vi "UHR-Fleezers Control (host) - 12.7d.vi"() -> ()   [LabVIEW 2012] (continued)
      }
      event "Load parameters": Value Change {
        n400 = event-data() -> ()  [unwired: 7 out]
        n401 = property on="Saved AOD Raster Scan Parameter Sets" class="Arr (strict)"() -> ("Index Values"=w577:u32[])  [unwired: 2 in, 2 out]
        n402 = Index Array(array=w577, index=0) -> (element=w574:u32)
        n403 = local write "Load parameters"(FALSE ("Load parameters")) -> ()
        n404 = Index Array(array="Saved AOD Raster Scan Parameter Sets", index=w574) -> (element=w573:T28)
        n405 = Unbundle By Name(w573) -> ("Scan Range AOD (nm) 2"=w572:dbl, "Step Size AOD (nm) 2"=w571:dbl, "Scan Speed AOD (nm/s) 2"=w570:dbl, "Number of scans (AOD) 2"=w569:u16)
        n406 = flat-sequence {
          tunnel: w572 -> [w580]
          tunnel: w571 -> [w579]
          tunnel: w570 -> [w578]
          tunnel: w569 -> [w581]
          frame #0 {
            n407 = local write "Scan Speed (nm/s)"(w578) -> ()
            n408 = local write "Scan Range (nm)"(w580) -> ()
            n409 = local write "Step Size (nm)"(w579) -> ()
          }
          frame #1 {
            n410 = property on="Number of F/B Scans (AOD)" class="DigNum (strict)"("Val(Sgnl)"=w581) -> ()  [unwired: 2 in, 2 out]
          }
        }
      }
      event "Trap 1 (ON/OFF)", "Trap 2 (ON/OFF)": Value Change {
        n411 = event-data() -> ()  [unwired: 7 out]
        n412 = property on="Trap 2 ON" class="Bool (strict)"("Val(Sgnl)"="Trap 2 (ON/OFF)") -> ()  [unwired: 2 in, 2 out]
        n413 = property on="Trap 1 ON" class="Bool (strict)"("Val(Sgnl)"="Trap 1 (ON/OFF)") -> ()  [unwired: 2 in, 2 out]
      }
      event "DIO count 1 (ticks)", "DIO count 2 (ticks)", "DIO count 3 (ticks)", "Interlace", "Number Interlace Sets", "Not-Interlacing Set", "BD 1 Delay (ticks)", "BD 2 Delay (Ticks)", "Next trap write delay (ticks)", "XY phase ext loop method", "Amp switch delay 2", "BD 2 Delay (Ticks) 2", "BD 1 Delay (ticks) 2": Value Change {
        n414 = event-data() -> ()  [unwired: 7 out]
        n415 = local read "DIO count 3 (ticks)"() -> (w602:u16)
        n416 = local read "DIO count 1 (ticks)"() -> (w604:u16)
        n417 = local read "DIO count 2 (ticks)"() -> (w603:u16)
        n418 = To Unsigned Byte Integer(number="Not-Interlacing Set") -> (unsigned 8bit integer=w593:u8)
        n419 = Add(x=w593, y=u8 1) -> (x+y=w597:u8)
        n420 = xnode "Read/Write Control"("FPGA VI Reference In"=w584, "DIO count 1 (ticks)"=w604, "DIO count 2 (ticks)"=w603, "DIO count 3 (ticks)"=w602, "Interlace ON/OFF"="Interlace", "Number Interlace Cycles"="Number Interlace Sets", "Interlace Off Parameters"=w597, "BD 1 Delay (ticks)"="BD 1 Delay (ticks)", "BD 2 Delay (Ticks)"="BD 2 Delay (Ticks)", "Next trap write delay (ticks)"="Next trap write delay (ticks)", "XY phase ext loop method"="XY phase ext loop method", "Amp switch delay 2"="Amp switch delay 2", "BD 2 Delay (Ticks) 2"="BD 2 Delay (Ticks) 2", "BD 1 Delay (ticks) 2"="BD 1 Delay (ticks) 2") -> ("error out"=w606:errorcluster)  [unwired: 1 in, 1 out]
        n421 = Build Array(w604, w603, w602) -> (w595:u16[])
        n422 = Split 1D Array(array=w595, index="Number Interlace Sets") -> (first subarray=w605:u16[])  [unwired: 1 out]
        n423 = Index Array(array=w595, index=w593) -> (element=w594:u16)
        n424 = Add Array Elements(numeric array=w605) -> (sum=w599:u16)
        n425 = Select(t=w599, s="Interlace", f=w594) -> (s? t:f=→"Total Counts (ticks)":u16)
      }
      event "Reset Feedback": Value Change {
        n426 = event-data() -> ()  [unwired: 7 out]
        n427 = Unbundle By Name("Reset Feedback") -> ("Set 1"=w610:bool, "Set 2"=w609:bool)
        n428 = xnode "Read/Write Control"("FPGA VI Reference In"=w607, "FB Reset Set 1"=w610, "FB Reset Set 2"=w609) -> ("error out"=w608:errorcluster)  [unwired: 1 in, 1 out]
      }
      event "Trap Intensity PID Gains": Value Change {
        n429 = event-data() -> ()  [unwired: 7 out]
        n430 = Unbundle By Name("Trap Intensity PID Gains") -> ("proportional gain (Kc)"=w615:i16, "integral gain (Kc*Ts/Ti)"=w614:i16, "derivative gain (Kc*Td/Ts)"=w613:i16)
        n431 = xnode "Read/Write Control"("FPGA VI Reference In"=w612, "P1"=w615, "I1"=w614, "D1"=w613) -> ("error out"=w617:errorcluster)  [unwired: 1 in, 1 out]
      }
      event "AI2 to Setpoint", "Setpoints (V)": Value Change {
        n432 = event-data() -> ()  [unwired: 7 out]
        n433 = xnode "Read/Write Control"("FPGA VI Reference In"=w618) -> ("FPGA VI Reference Out"=w621:T20, "error out"=w620:errorcluster, "AI2 Y Sum Set 1"=w628:i16, "AI2 Y Sum Set 2"=w627:i16)  [unwired: 1 in]
        n434 = Cluster To Array(cluster="AI2 to Setpoint") -> (array=w631:bool[])
        n435 = local read "AI2 (V)"() -> (w629:cluster{"Set 1":dbl, "Set 2":dbl})
        n436 = Or Array Elements(Boolean array=w631) -> (logical OR=w632:bool)
        n437 = Bundle By Name(cluster=w629, "Set 1"=w628, "Set 2"=w627) -> (w626:cluster{"Set 1":dbl, "Set 2":dbl})
        n438 = Divide(x=w626, y=3276.7) -> (x/y=w625:cluster{"Set 1":dbl, "Set 2":dbl})
        "AI2 (V)" <- w625
        n439 = case shown="True" w632 {
          tunnel: [w635 w652] -> w624
          tunnel: "AI2 to Setpoint" -> [_ w648]
          tunnel: "Setpoints (V)" -> [w636 w651]
          tunnel: w625 -> [_ w645]
          frame False {
            n440 = Multiply(x=3276.7, y=w636) -> (x*y=w637:cluster{"Set 1":dbl, "Set 2":dbl})
            n441 = To Word Integer(number=w637) -> (16bit integer=w635:cluster{"Set 1":i16, "Set 2":i16})
          }
          frame True {
            n442 = Unbundle By Name(w645) -> ("Set 1"=w644:dbl, "Set 2"=w643:dbl)
            n443 = Unbundle By Name(w651) -> ("Set 1"=w650:dbl, "Set 2"=w649:dbl)
            n444 = Unbundle By Name(w648) -> ("Set 1"=w647:bool, "Set 2"=w646:bool)
            n445 = Select(t=w644, s=w647, f=w650) -> (s? t:f=w642:dbl)
            n446 = Select(t=w643, s=w646, f=w649) -> (s? t:f=w641:dbl)
            n447 = Bundle By Name(cluster=w651, "Set 1"=w642, "Set 2"=w641) -> (w639:cluster{"Set 1":dbl, "Set 2":dbl})
            n448 = local write "Setpoints (V)"(w639) -> ()
            n449 = Multiply(x=3276.7, y=w639) -> (x*y=w640:cluster{"Set 1":dbl, "Set 2":dbl})
            n450 = To Word Integer(number=w640) -> (16bit integer=w652:cluster{"Set 1":i16, "Set 2":i16})
          }
        }
        n451 = Unbundle By Name(w624) -> ("Set 1"=w623:i16, "Set 2"=w622:i16)
        n452 = xnode "Read/Write Control"("FPGA VI Reference In"=w621, "error in"=w620, "FB Setpoint Set 1"=w623, "FB Setpoint Set 2"=w622) -> ("error out"=w619:errorcluster)  [unwired: 1 out]
      }
      event "+ phase (GI)", "- phase (GI)", "+ phase (GI) 2", "- phase (GI) 2", "+ phase (RI)", "- phase (RI)", "+ phase (Green FB)", "- phase (Green FB)": Value Change {
        n453 = event-data() -> ()  [unwired: 7 out]
        n454 = Or(x="+ phase (GI)", y="- phase (GI)") -> (x .or. y?=w688:bool)
        n455 = Negate(x="Phase adj. (GI)") -> (-x=w693:i16)
        n456 = Select(t=w693, s="+ phase (GI)", f="Phase adj. (GI)") -> (s? t:f=w692:i16)
        n457 = Or(x="+ phase (GI) 2", y="- phase (GI) 2") -> (x .or. y?=w679:bool)
        n458 = Negate(x="Phase adj. (GI) 2") -> (-x=w684:i16)
        n459 = Select(t=w684, s="+ phase (GI) 2", f="Phase adj. (GI) 2") -> (s? t:f=w680:i16)
        n460 = Negate(x="Phase adj. (RI)") -> (-x=w678:i16)
        n461 = Or(x="+ phase (RI)", y="- phase (RI)") -> (x .or. y?=w674:bool)
        n462 = Select(t=w678, s="+ phase (RI)", f="Phase adj. (RI)") -> (s? t:f=w673:i16)
        n463 = Or(x="+ phase (Green FB)", y="- phase (Green FB)") -> (x .or. y?=w667:bool)
        n464 = Negate(x="Phase adj. (Green FB)") -> (-x=w672:i16)
        n465 = Select(t=w672, s="+ phase (Green FB)", f="Phase adj. (Green FB)") -> (s? t:f=w668:i16)
        n466 = Negate(x="Phase adj. (BI AO)") -> (-x=w666:i16)
        n467 = Or(x="+ phase (BI AO)", y="- phase (BI AO)") -> (x .or. y?=w656:bool)
        n468 = Select(t=w666, s="+ phase (BI AO)", f="Phase adj. (BI AO)") -> (s? t:f=w658:i16)
        n469 = Negate(x="Phase adj. (BI DO)") -> (-x=w662:i16)
        n470 = Or(x="+ phase (BI DO)", y="- phase (BI DO)") -> (x .or. y?=w655:bool)
        n471 = Select(t=w662, s="+ phase (BI DO)", f="Phase adj. (BI DO)") -> (s? t:f=w657:i16)
        n472 = xnode "Read/Write Control"("FPGA VI Reference In"=w654, "Phase count adjustment (GI)"=w692, "Phase count adjustment (GI) 2"=w680, "Phase count adjustment (RI)"=w673, "Phase count adjustment (Green FB)"=w668, "Phase count adjustment (BI AO)"=w658, "Phase count adjustment (BI D)"=w657) -> ("FPGA VI Reference Out"=w690:T20, "error out"=w691:errorcluster)  [unwired: 1 in]
        n473 = xnode "Read/Write Control"("FPGA VI Reference In"=w690, "error in"=w691, "+ phase (GI)"=w688, "+ phase (GI) 2"=w679, "+ phase (RI)"=w674, "+ phase (Green FB)"=w667, "+ phase (BI AO)"=w656, "+ phase (BI D)"=w655) -> ("error out"=w689:errorcluster)  [unwired: 1 out]
      }
      event "Green Laser ON/OFF", "Red Laser ON/OFF", "Blue Laser ON/OFF": Value Change {
        # "This loop shouldn't be initialized.  The main 'laser ON' settings should dominate and set the others."
        n474 = event-data() -> ()  [unwired: 7 out]
        n475 = property on="Red Laser ON" class="Bool (strict)"("Val(Sgnl)"="Red Laser ON/OFF") -> ()  [unwired: 2 in, 2 out]
        n476 = property on="Blue Laser ON" class="Bool (strict)"("Val(Sgnl)"="Blue Laser ON/OFF") -> ()  [unwired: 2 in, 2 out]
        n477 = property on="Green Laser ON" class="Bool (strict)"("Val(Sgnl)"="Green Laser ON/OFF") -> ()  [unwired: 2 in, 2 out]
      }
      event "Laser interlacing mode", "Green Laser ON", "Red Laser ON", "Blue Laser ON": Value Change {
        n478 = event-data() -> ()  [unwired: 7 out]
        n479 = local write "Green Laser ON/OFF"("Green Laser ON") -> ()
        n480 = local write "Blue Laser ON/OFF"("Blue Laser ON") -> ()
        n481 = local write "Red Laser ON/OFF"("Red Laser ON") -> ()
        n482 = case shown="True" "Green Laser ON" {
          tunnel: "Laser interlacing mode" -> [_ w729]
          tunnel: [enum32{"Laser ON", "Laser OFF", "Interlace"}."Laser OFF" ("Green laser mode") w729] -> w707
          tunnel: [FALSE w725] -> w706
          frame False {
          }
          frame True {
            n483 = local read "Green FB On/Off"() -> (w726:bool)
            n484 = Equal?(x=w729, y=enum32{"Laser ON", "Laser OFF", "Interlace"}."Interlace") -> (x = y?=w727:bool)
            n485 = And(x=w727, y=w726) -> (x .and. y?=w725:bool)
          }
        }
        n486 = case shown="True" "Red Laser ON" {
          tunnel: "Laser interlacing mode" -> [_ w722]
          tunnel: [enum32{"Laser ON", "Laser OFF", "Interlace"}."Laser OFF" ("Green laser mode") w722] -> w703
          tunnel: [FALSE w718] -> w702
          frame False {
          }
          frame True {
            n487 = local read "Red FB On/Off"() -> (w719:bool)
            n488 = Equal?(x=w722, y=enum32{"Laser ON", "Laser OFF", "Interlace"}."Interlace") -> (x = y?=w720:bool)
            n489 = And(x=w720, y=w719) -> (x .and. y?=w718:bool)
          }
        }
        n490 = case shown="True" "Blue Laser ON" {
          tunnel: "Laser interlacing mode" -> [_ w713]
          tunnel: [enum32{"Laser ON", "Laser OFF", "Interlace"}."Laser OFF" ("Green laser mode") w713] -> w699
          tunnel: [FALSE w711] -> w698
          frame False {
          }
          frame True {
            n491 = local read "Blue FB On/Off"() -> (w712:bool)
            n492 = Equal?(x=w713, y=enum32{"Laser ON", "Laser OFF", "Interlace"}."Interlace") -> (x = y?=w714:bool)
            n493 = And(x=w714, y=w712) -> (x .and. y?=w711:bool)
          }
        }
        n494 = xnode "Read/Write Control"("FPGA VI Reference In"=w697, "Operating Mode"=w707, "Operating Mode 2"=w707, "Green FB On/Off"=w706, "Red Laser Operating Mode"=w703, "RI Operating Mode 2"=w703, "Red FB On/Off"=w702, "BI Operating Mode (AO)"=w699, "Blue Laser Operating Mode (D)"=w699, "Blue FB On/Off"=w698) -> ("error out"=w708:errorcluster)  [unwired: 1 in, 1 out]
      }
      event "Invert laser interlacing": Value Change {
        n495 = event-data() -> ()  [unwired: 7 out]
        n496 = xnode "Read/Write Control"("FPGA VI Reference In"=w730, "Invert GI"="Invert laser interlacing", "Invert GI 2"="Invert laser interlacing", "Invert RI"="Invert laser interlacing", "Invert RI 2"="Invert laser interlacing", "Invert BI (AO)"="Invert laser interlacing", "Invert BI (D)"="Invert laser interlacing") -> ("error out"=w732:errorcluster)  [unwired: 1 in, 1 out]
      }
      event "Green FB Setpoint (mV)", "Green FB Gains", "Green FB On/Off", "Green Intensity % (FB OFF)", "Green int current ON count adj": Value Change {
        n497 = event-data() -> ()  [unwired: 7 out]
        n498 = local read "Green FB Setpoint (mV)"() -> (w744:dbl)
        n499 = Multiply(x=w744, y=3.2767) -> (x*y=w743:dbl)
        n500 = local read "Green Intensity % (FB OFF)"() -> (w747:dbl)
        n501 = Multiply(x=w747, y=655.35) -> (x*y=w748:dbl)
        n502 = To Unsigned Word Integer(number=w748) -> (unsigned 16bit integer=w746:u16)
        n503 = local read "Green int current ON count adj"() -> (w750:u32)
        n504 = local read "Laser interlacing mode"() -> (w740:enum32{"Laser ON", "Laser OFF", "Interlace"})
        n505 = local read "Green FB Gains"() -> (w737:T9)
        n506 = local read "Green Laser ON"() -> (w741:bool)
        n507 = local read "Green FB On/Off"() -> (w751:bool)
        n508 = Equal?(x=w740, y=enum32{"Laser ON", "Laser OFF", "Interlace"}."Interlace") -> (x = y?=w738:bool)
        n509 = Unbundle By Name(w737) -> ("proportional gain (Kc)"=w736:i16, "integral gain (Kc*Ts/Ti)"=w735:i16, "derivative gain (Kc*Td/Ts)"=w734:i16)
        n510 = Compound Arithmetic op=AND(w738, w751, w741) -> (w742:bool)
        n511 = xnode "Read/Write Control"("FPGA VI Reference In"=w733, "Green FB Setpoint"=w743, "Green FB On/Off"=w742, "Current Out"=w746, "Green int current ON count adj"=w750, "P3"=w736, "I3"=w735, "D3"=w734) -> ("error out"=w752:errorcluster)  [unwired: 1 in, 1 out]
      }
      event "Blue FB Setpoint (mV)", "Blue FB Gains", "Blue FB On/Off", "Blue Intensity % (FB OFF)", "Blue int AO ON count adjust": Value Change {
        # "16 bit analog out"
        n512 = event-data() -> ()  [unwired: 7 out]
        n513 = Multiply(x="Blue FB Setpoint (mV)", y=3.2767) -> (x*y=w767:dbl)
        n514 = Multiply(x="Blue Intensity % (FB OFF)", y=655.35) -> (x*y=w770:dbl)
        n515 = To Unsigned Word Integer(number=w770) -> (unsigned 16bit integer=w769:u16)
        n516 = local read "Laser interlacing mode"() -> (w765:enum32{"Laser ON", "Laser OFF", "Interlace"})
        n517 = Unbundle By Name("Blue FB Gains") -> ("proportional gain (Kc)"=w762:i16, "integral gain (Kc*Ts/Ti)"=w761:i16, "derivative gain (Kc*Td/Ts)"=w760:i16)
        n518 = local read "Blue Laser ON"() -> (w754:bool)
        n519 = Equal?(x=w765, y=enum32{"Laser ON", "Laser OFF", "Interlace"}."Interlace") -> (x = y?=w763:bool)
        n520 = Compound Arithmetic op=AND(w763, "Blue FB On/Off", w754) -> (w766:bool)
        n521 = xnode "Read/Write Control"("FPGA VI Reference In"=w753, "Blue FB Setpoint"=w767, "Blue FB On/Off"=w766, "BI Current Out"=w769, "Blue current ON count adj (AO)"="Blue int AO ON count adjust", "P5"=w762, "I5"=w761, "D5"=w760) -> ("error out"=w772:errorcluster)  [unwired: 1 in, 1 out]
      }
      event "Red FB Setpoint (mV)", "Red FB Gains", "Red FB On/Off", "Red Intensity % (FB OFF)": Value Change {
        n522 = event-data() -> ()  [unwired: 7 out]
        n523 = local read "Red FB Setpoint (mV)"() -> (w785:dbl)
        n524 = Multiply(x=w785, y=3.2767) -> (x*y=w784:dbl)
        n525 = local read "Red Intensity % (FB OFF)"() -> (w774:dbl)
        n526 = Multiply(x=w774, y=655.35) -> (x*y=w788:dbl)
        n527 = To Unsigned Word Integer(number=w788) -> (unsigned 16bit integer=w787:u16)
        n528 = local read "Laser interlacing mode"() -> (w781:enum32{"Laser ON", "Laser OFF", "Interlace"})
        n529 = local read "Red FB Gains"() -> (w778:T9)
        n530 = local read "Red Laser ON"() -> (w782:bool)
        n531 = local read "Red FB On/Off"() -> (w790:bool)
        n532 = Equal?(x=w781, y=enum32{"Laser ON", "Laser OFF", "Interlace"}."Interlace") -> (x = y?=w779:bool)
        n533 = Unbundle By Name(w778) -> ("proportional gain (Kc)"=w777:i16, "integral gain (Kc*Ts/Ti)"=w776:i16, "derivative gain (Kc*Td/Ts)"=w775:i16)
        n534 = Compound Arithmetic op=AND(w779, w790, w782) -> (w783:bool)
        n535 = xnode "Read/Write Control"("FPGA VI Reference In"=w773, "Red FB Setpoint"=w784, "Red FB On/Off"=w783, "RI Current Out"=w787, "P4"=w777, "I4"=w776, "D4"=w775) -> ("error out"=w791:errorcluster)  [unwired: 1 in, 1 out]
      }
      event "+ phase (APD 1 Gate)", "- phase (APD 1 Gate)", "+ phase (APD 2 Gate)", "- phase (APD 2 Gate)", "+ phase (APD 3 Gate)", "- phase (APD 3 Gate)", "+ phase (APD Acq)", "- phase (APD Acq)": Value Change {
        n536 = event-data() -> ()  [unwired: 7 out]
        n537 = local read "Phase Adj. (APD 1 Gate)"() -> (w812:i16)
        n538 = Or(x="- phase (APD 1 Gate)", y="+ phase (APD 1 Gate)") -> (x .or. y?=w814:bool)
        n539 = Negate(x=w812) -> (-x=w819:i16)
        n540 = Select(t=w819, s="+ phase (APD 1 Gate)", f=w812) -> (s? t:f=w818:i16)
        n541 = local read "Phase Adj. (APD 2 Gate)"() -> (w809:i16)
        n542 = Or(x="- phase (APD 2 Gate)", y="+ phase (APD 2 Gate)") -> (x .or. y?=w807:bool)
        n543 = Negate(x=w809) -> (-x=w811:i16)
        n544 = Select(t=w811, s="+ phase (APD 2 Gate)", f=w809) -> (s? t:f=w808:i16)
        n545 = Negate(x="Phase Adj. (APD 3 Gate)") -> (-x=w806:i16)
        n546 = Or(x="- phase (APD 3 Gate)", y="+ phase (APD 3 Gate)") -> (x .or. y?=w802:bool)
        n547 = Select(t=w806, s="+ phase (APD 3 Gate)", f="Phase Adj. (APD 3 Gate)") -> (s? t:f=w803:i16)
        n548 = local read "Phase Adj. (APD Acq)"() -> (w800:i16)
        n549 = Or(x="- phase (APD Acq)", y="+ phase (APD Acq)") -> (x .or. y?=w798:bool)
        n550 = Negate(x=w800) -> (-x=w801:i16)
        n551 = Select(t=w801, s="+ phase (APD Acq)", f=w800) -> (s? t:f=w799:i16)
        n552 = xnode "Read/Write Control"("FPGA VI Reference In"=w792, "Phase count adjustment (APD 1 Gate)"=w818, "Phase count adjustment (APD 2 Gate)"=w808, "Phase count adjustment (APD 3 Gate)"=w803, "Phase Count Adjustment (APD Acq)"=w799) -> ("FPGA VI Reference Out"=w816:T20, "error out"=w817:errorcluster)  [unwired: 1 in]
        n553 = xnode "Read/Write Control"("FPGA VI Reference In"=w816, "error in"=w817, "+ phase (APD 1 Gate)"=w814, "+ phase (APD 2 Gate)"=w807, "+ phase (APD 3 Gate)"=w802, "+ phase (APD Acq)"=w798) -> ("error out"=w815:errorcluster)  [unwired: 1 out]
      }
      event "Invert APD Gate", "APD Gate ON Count", "APD Gate OFF Count", "APD Gate", "APD Integration Time (s)", "APD AO Scale Factor", "Duty Frequency (ON 1/N cycles)", "Interlace ON count", "Interlace OFF count": Value Change {
        n554 = event-data() -> ()  [unwired: 7 out]
        n555 = Add(x="Interlace ON count", y="Interlace OFF count") -> (x+y=w826:u16)
        n556 = Add(x="APD Gate ON Count", y="APD Gate OFF Count") -> (x+y=w837:u16)
        n557 = Multiply(x="Duty Frequency (ON 1/N cycles)", y=w826) -> (x*y=w822:u16)
        "Green AI Count" <- w822
        "Red AI Count" <- w822
        "Blue AI Count" <- w822
        n558 = Subtract(x=w822, y="Interlace ON count") -> (x-y=w825:u16)
        n559 = Multiply(x=w837, y="Duty Frequency (ON 1/N cycles)") -> (x*y=w836:u16)
        n560 = Subtract(x=w836, y="APD Gate ON Count") -> (x-y=w835:u16)
        n561 = local read "DMA Update Period (s)"() -> (w838:dbl)
        n562 = Multiply(x="APD Integration Time (s)", y=40000000.0) -> (x*y=w842:dbl)
        n563 = Reciprocal(x="APD Integration Time (s)") -> (1/x=→"APD Acq Rate (Hz)":dbl)
        n564 = To Unsigned Long Integer(number=w842) -> (unsigned 32bit integer=w828:u32)
        "APD Int. Count" <- w828
        n565 = local read "Number of APDs"() -> (w821:u8)
        n566 = Divide(x=w838, y="APD Integration Time (s)") -> (x/y=w840:dbl)
        n567 = Multiply(x=w821, y=w840) -> (x*y=w839:dbl)
        n568 = local write "APD Samples/FIFO Acq."(w840) -> ()
        n569 = local write "APD Elements/DMA read"(w839) -> ()
        n570 = xnode "Read/Write Control"("FPGA VI Reference In"=w820, "Invert APD Gate"="Invert APD Gate", "APD Gate ON Count"="APD Gate ON Count", "APD Gate OFF Count"=w835, "APD Acq Rate Count"=w828, "APD Gate Operating Mode"="APD Gate", "APD AO scale factor"="APD AO Scale Factor", "Green interlace ON count"="Interlace ON count", "Green interlace OFF count"=w825, "Green interlace ON count 2"="Interlace ON count", "Green interlace OFF count 2"=w825, "Green FB Count"=w822, "Red interlace ON count"="Interlace ON count", "Red interlace OFF count"="Interlace OFF count", "Blue ON count (AO)"="Interlace ON count", "Blue OFF count (AO)"="Interlace OFF count", "Blue interlace OFF count (D)"="Interlace OFF count", "Blue interlace ON count (D)"="Interlace ON count") -> ("error out"=w844:errorcluster)  [unwired: 1 in, 1 out]
      }
      event "Neg. TTrig FPGA": Value Change {
        n571 = event-data() -> ()  [unwired: 7 out]
        n572 = xnode "Read/Write Control"("FPGA VI Reference In"=w845, "TTrig Negate Pos"="Neg. TTrig FPGA") -> ()  [unwired: 1 in, 2 out]
      }
      event "Test ttrig": Value Change {
        n573 = event-data() -> ()  [unwired: 7 out]
        n574 = xnode "Read/Write Control"("FPGA VI Reference In"=w847, "TTrig?"=TRUE) -> ("error out"=w849:errorcluster)  [unwired: 1 in, 1 out]
      }
      event "Number of F/B Scans (AOD)", "Scan Speed (nm/s)", "Scan BD", "Initial delta (MHz)", "Step Size (nm)", "Scan Range (nm)": Value Change {
        w913 = 123.0  # AOM cal (nm/MHz)
        n575 = event-data() -> ()  [unwired: 7 out]
        n576 = local read "BD 1 Frequency 1 (MHz)"() -> (w896:dbl)
        n577 = local read "AOM X Cal (nm/MHz)"() -> (w888:dbl)
        n578 = local read "X RF Frequency Limits (MHz)"() -> (w900:T16)
        n579 = local read "Y RF Frequency Limits (MHz)"() -> (w897:T16)
        n580 = local read "BD 2 Frequency 1 (MHz)"() -> (w902:dbl)
        n581 = Negate(x="Scan Range (nm)") -> (-x=w866:dbl)
        n582 = Divide(x=w866, y=w888) -> (x/y=w870:dbl)
        n583 = Select(t=w900, s="Scan BD", f=w897) -> (s? t:f=w899:T16)
        n584 = Select(t=w896, s="Scan BD", f=w902) -> (s? t:f=w901:dbl)
        n585 = Unbundle By Name(w899) -> ("Maximum"=w908:dbl, "Minimum"=w907:dbl)
        n586 = Add(x=w870, y=w901) -> (x+y=w905:dbl)
        n587 = Divide(x=w866, y="Step Size (nm)") -> (x/y=w885:dbl)
        n588 = Divide(x="Step Size (nm)", y=w888) -> (x/y=w894:dbl)
        n589 = Absolute Value(x=w885) -> (abs(x)=w869:dbl)
        n590 = Sign(1:w866) -> (0:w867:dbl)
        n591 = In Range and Coerce(upper limit=w908, x=w905, lower limit=w907) -> (coerced(x)=w904:dbl, In Range?=w906:bool)
        n592 = To Unsigned Quad Integer(1:w869) -> (0:w884:u64)
        "Scan steps (AOD)" <- w884
        n593 = call "IR AOM freq to word.vi"("Frequency In (MHz)"=w894) -> ("Frequency Word Out (double)"=w891:dbl)
        n594 = Multiply(x=w867, y=w891) -> (x*y=w868:dbl)
        n595 = Subtract(x=w905, y=w904) -> (x-y=w903:dbl)
        n596 = To Quad Integer(1:w868) -> (0:w890:i64)
        "Incr. int (AOD)" <- w890
        n597 = Subtract(x=w870, y=w903) -> (x-y=w889:dbl)
        "Scan Range (MHz)" <- w889
        n598 = Select(t=w870, s=w906, f=w889) -> (s? t:f=w909:dbl)
        n599 = Multiply(x=w889, y=w888) -> (x*y=w887:dbl)
        n600 = Decrement(x=w884) -> (x-1=w937:u64)
        n601 = Negate(x=w887) -> (-x=w883:dbl)
        n602 = local write "Scan Range (nm)"(w883) -> ()
        n603 = Divide(x=w909, y=w937) -> (x/y=w893:dbl)
        "Scan Increment (MHz)" <- w893
        n604 = call "IR AOM freq to word.vi"("Frequency In (MHz)"=w893) -> ("Frequency Word Out (double)"=w892:dbl)
        n605 = Divide(x="Step Size (nm)", y="Scan Speed (nm/s)") -> (x/y=w880:dbl)
        n606 = To Quad Integer(1:w892) -> ()  [unwired: 1 out]
        n607 = local read "Number Interlace Sets"() -> (w864:u8)
        n608 = local read "AI Count (ticks)"() -> (w865:u16)
        n609 = local read "Total Counts (ticks)"() -> (w863:u16)
        n610 = local read "# Samples/trap"() -> (w895:u32)
        n611 = Multiply(x=w865, y=w864) -> (x*y=w862:u16)
        n612 = Divide(x=w863, y=w862) -> (x/y=w861:dbl)
        n613 = Select(t=w896, s="Scan BD", f=w902) -> (s? t:f=w934:dbl)
        "Initial freq. (MHz)" <- w934
        n614 = Add(x=w909, y=w934) -> (x+y=→"Final freq. (MHz)":dbl)
        n615 = Divide(x=w863, y=40000000.0) -> (x/y=w879:dbl)
        n616 = Divide(x=w880, y=w879) -> (x/y=w878:dbl)
        n617 = To Unsigned Quad Integer(1:w878) -> (0:w853:u64)
        n618 = Quotient & Remainder(x=w853, y=u64 2) -> (x-y*floor(x/y)=w857:u64)  [unwired: 1 out]
        n619 = Equal?(x=w857, y=u64 0) -> (x = y?=w855:bool)
        n620 = Decrement(x=w853) -> (x-1=w854:u64)
        n621 = Select(t=w853, s=w855, f=w854) -> (s? t:f=w852:u64)
        "Cycles/step (AOD)" <- w852
        n622 = xnode "Read/Write Control"("FPGA VI Reference In"=w851, "Scan steps"=w884, "Number of scans"="Number of F/B Scans (AOD)", "Cycles per step"=w852, "Scan freq.  increment"=w890, "Scan BD"="Scan BD") -> ("error out"=w943:errorcluster)  [unwired: 1 in, 1 out]
        n623 = Multiply(x=w884, y=w852) -> (x*y=w938:u64)
        n624 = Multiply(x=w938, y=u64 2) -> (x*y=w860:u64)
        n625 = Multiply(x=w861, y=w860) -> (x*y=w859:dbl)
        "Data points/scan (f/b)" <- w859
        n626 = Multiply(x=w859, y="Number of F/B Scans (AOD)") -> (x*y=w941:dbl)
        "Data points/scans" <- w941
        n627 = Divide(x=w941, y=w895) -> (x/y=→"N sets should be saved":dbl)
        n628 = Multiply(x=w938, y=w879) -> (x*y=w877:dbl)
        "Time/Scan (s) (AOD)" <- w877
        n629 = Select(t=w909, s="Scan BD", f=0.0) -> (s? t:f=w935:dbl)
        n630 = Select(t=0.0, s="Scan BD", f=w909) -> (s? t:f=w931:dbl)
        n631 = local read "BD 2 Frequency 2 (MHz)"() -> (w927:dbl)
        n632 = local read "BD 1 Frequency 2 (MHz)"() -> (w930:dbl)
        n633 = Add(x=w931, y=w902) -> (x+y=w928:dbl)
        n634 = Add(x=w896, y=w935) -> (x+y=w929:dbl)
        n635 = Multiply(x=w877, y=2.0) -> (x*y=w876:dbl)
        n636 = Multiply(x=w876, y="Number of F/B Scans (AOD)") -> (x*y=w873:dbl)
        n637 = Divide(x=w873, y=60.0) -> (x/y=→"Time to Finish All (min)":dbl)
        n638 = Add(x="Trap 2 Bead Size (nm)", y="Trap 1 Bead Size (nm)") -> (x+y=w917:dbl)
        n639 = Divide(x=w917, y=2.0) -> (x/y=w911:dbl)
        n640 = local read "Initial delta (MHz)"() -> (w914:dbl)
        n641 = Subtract(x=w928, y=w927) -> (x-y=w925:dbl)
        n642 = Subtract(x=w929, y=w930) -> (x-y=w926:dbl)
        n643 = Square(x=w925) -> (x^2=w924:dbl)
        n644 = Square(x=w926) -> (x^2=w923:dbl)
        n645 = Add(x=w923, y=w924) -> (x+y=w922:dbl)
        n646 = Square Root(x=w922) -> (sqrt(x)=w921:dbl)
        "Final delta (MHz)" <- w921
        n647 = Multiply(x=w913, y=w921) -> (x*y=w920:dbl)
        n648 = Multiply(x=w914, y=w913) -> (x*y=w912:dbl)
        n649 = Subtract(x=w912, y=w911) -> (x-y=→"Initial sep (nm)":dbl)
        n650 = Subtract(x=w920, y=w911) -> (x-y=→"Final sep (nm)":dbl)
      }
      event "Freq or Amp switch first", "Swap F1 and F2", "Freq switch delay", "Amp switch delay": Value Change {
        n651 = event-data() -> ()  [unwired: 7 out]
        n652 = local read "Amp switch delay"() -> (w945:u16)
        n653 = local read "Swap F1 and F2"() -> (w946:bool)
        n654 = xnode "Read/Write Control"("FPGA VI Reference In"=w944, "Swap F1 and F2"=w946, "Amp switch delay"=w945) -> ("error out"=w947:errorcluster)  [unwired: 1 in, 1 out]
      }
      event "Scan steps (MCL)", "Number of scans (MCL)", "Scan Range (V)\n(of steps)", "2D or 1D Scan", "N APD Samp/step", "Fast Scan Dir", "Continuous MCL Scanning", "Scan lines (y)": Value Change {
        w950 = 32767.0 ("y")
        n655 = event-data() -> ()  [unwired: 7 out]
        n656 = Select(t="Scan lines (y)", s="2D or 1D Scan", f="Number of scans (MCL)") -> (s? t:f=w955:u64)
        n657 = Decrement(x="Scan steps (MCL)") -> (x-1=w971:u64)
        n658 = Divide(x="Scan Range (V)\n(of steps)", y=w971) -> (x/y=w970:dbl)
        "Desired Scan Incr (V)" <- w970
        n659 = local read "APD Integration Time (s)"() -> (w963:dbl)
        n660 = Multiply(x=w970, y=w950) -> (x*y=w979:dbl)
        n661 = Divide(x=w979, y=10.0) -> (x/y=w969:dbl)
        "Desired incr (int)" <- w969
        n662 = local read "Update Count (MCL)"() -> (w975:u32)
        n663 = Round Toward -Infinity(1:w969) -> (0:w978:dbl)
        n664 = To Word Integer(number=w978) -> (16bit integer=w953:i16)
        "Actual Incr. int (MCL)" <- w953
        n665 = Multiply(x=w963, y=40000000.0) -> (x*y=w976:dbl)
        n666 = Divide(x=w976, y=w975) -> (x/y=w974:dbl)
        n667 = Multiply(x=i16 10, y=w953) -> (x*y=w951:i16)
        n668 = Multiply(x="N APD Samp/step", y=w974) -> (x*y=w973:dbl)
        "Cycles/step (MCL)" <- w973
        n669 = Divide(x=w951, y=w950) -> (x/y=→"Actual MCL Inc (V)":dbl)
        n670 = Multiply(x="N APD Samp/step", y="Scan steps (MCL)") -> (x*y=w965:dbl)
        n671 = local read "APD Samples/FIFO Acq."() -> (w962:dbl)
        n672 = Multiply(x=w965, y=u64 2) -> (x*y=w964:dbl)
        "Data points/scan (f+b)" <- w964
        n673 = Multiply(x=w964, y=w955) -> (x*y=w982:dbl)
        "Data points/scans (MCL)" <- w982
        n674 = Multiply(x=w963, y=w964) -> (x*y=w956:dbl)
        "Time/f+b scan (s) (MCL)" <- w956
        n675 = Divide(x=w982, y=w962) -> (x/y=→"N sets should be saved (MCL)":dbl)
        n676 = Multiply(x=w956, y=w955) -> (x*y=→"Total Time (s)":dbl)
        n677 = Not(x="Fast Scan Dir") -> (.not. x?=w960:bool)
        n678 = xnode "Read/Write Control"("FPGA VI Reference In"=w948, "Scan steps (MCL)"="Scan steps (MCL)", "Number of scans (MCL)"=w955, "Cycles per step (MCL)"=w973, "Scan freq.  increment (MCL)"=w953, "1D or 2D Scan?"="2D or 1D Scan", "MCL Scan Axis"=w960, "Cont. Scan (MCL)"="Continuous MCL Scanning") -> ("error out"=w984:errorcluster)  [unwired: 1 in, 1 out]
      }
      event "Read Cal": Value Change {
        w986 = 1000.0 ("y")
        n679 = event-data() -> ()  [unwired: 7 out]
        n680 = local read "Save file name"() -> (w1011:path)
        n681 = local write "Read Cal"(FALSE ("Read Cal")) -> ()
        n682 = Strip Path(path=w1011) -> (stripped path=w1010:path)  [unwired: 1 out]
        n683 = Path To String(path=w1010) -> (string=w1009:string)
        n684 = Concatenate Strings(w1009, "\\current.cal" ("string")) -> (w1007:string)
        n685 = String To Path(string=w1007) -> (path=w1006:path)
        n686 = Open/Create/Replace File(file path (use dialog)=w1006, operation (0:open)=T27."open", access (0:read/write)=enum16{"read/write", "read-only", "write-only"}."read-only") -> (refnum out=w1014:refnum<file>, error out=w1000:errorcluster)  [unwired: 1 in, 3 out]
        n687 = Deny Access(4:w1000, 7:w1014) -> (0:w999:errorcluster, 3:w1005:refnum<file>)  [unwired: 1 out]
        n688 = Read from Binary File(5:0.0, 8:w999, 9:T26."big-endian, network order" ("byte order (0:big-endian, network order)"), 10:-1 ("count (1)"), 11:w1005) -> (0:w998:errorcluster, 2:w996:dbl[], 3:w1001:refnum<file>)  [unwired: 2 out]
        n689 = Array To Cluster(array=w996) -> (cluster=w995:T29)
        n690 = Unbundle(w995) -> ("[0]"=w994:dbl, "[1]"=w993:dbl, "[2]"=w992:dbl, "[3]"=w991:dbl, "[4]"=w990:dbl, "[5]"=w989:dbl)
        n691 = Close File(refnum=w1001, error in=w998) -> (error out=→"Read cal error":errorcluster)  [unwired: 1 out]
        n692 = Multiply(x=w989, y=w986) -> (x*y=w987:dbl)
        n693 = local write "T2 kappa_x (pN/nm)"(w991) -> ()
        n694 = local write "T1 kappa_x (pN/nm)"(w992) -> ()
        n695 = local write "T1 alpha_x (nm/V)"(w994) -> ()
        n696 = local write "T2 alpha_x (nm/V)"(w993) -> ()
        n697 = Multiply(x=w990, y=w986) -> (x*y=w988:dbl)
        n698 = local write "T1 offset_x (mV)"(w988) -> ()
        n699 = local write "T2 offset_x (mV)"(w987) -> ()
      }
      event "Abort MCL Scan": Value Change {
        n700 = event-data() -> ()  [unwired: 7 out]
        n701 = local write "MCL Scanning"(FALSE ("MCL Scanning")) -> ()
        n702 = xnode "Read/Write Control"("FPGA VI Reference In"=w1015, "Abort scan (MCL)"="Abort MCL Scan") -> ("error out"=w1018:errorcluster)  [unwired: 1 in, 1 out]
      }
      event "Update Count (MCL)": Value Change {
        n703 = event-data() -> ()  [unwired: 7 out]
        n704 = xnode "Read/Write Control"("FPGA VI Reference In"=w1019, "MCL count"="Update Count (MCL)") -> ("error out"=w1021:errorcluster)  [unwired: 1 in, 1 out]
      }
      event "+ phase (MCL)", "- phase (MCL)": Value Change {
        n705 = event-data() -> ()  [unwired: 7 out]
        n706 = Or(x="- phase (MCL)", y="+ phase (MCL)") -> (x .or. y?=w1025:bool)
        n707 = Negate(x="Phase adjust (MCL)") -> (-x=w1031:i16)
        n708 = Select(t=w1031, s="+ phase (MCL)", f="Phase adjust (MCL)") -> (s? t:f=w1029:i16)
        n709 = xnode "Read/Write Control"("FPGA VI Reference In"=w1022, "Phase count adjustment (MCL)"=w1029) -> ("FPGA VI Reference Out"=w1026:T20, "error out"=w1027:errorcluster)  [unwired: 1 in]
        n710 = xnode "Read/Write Control"("FPGA VI Reference In"=w1026, "error in"=w1027, "+ phase (MCL)"=w1025) -> ("error out"=w1024:errorcluster)  [unwired: 1 out]
      }
      event "Abort AOD Scan": Value Change {
        n711 = event-data() -> ()  [unwired: 7 out]
        n712 = xnode "Read/Write Control"("FPGA VI Reference In"=w1032, "Abort scan"="Abort AOD Scan") -> ("error out"=w1034:errorcluster)  [unwired: 1 in, 1 out]
      }
      event "Continuous AOD Scanning": Value Change {
        n713 = event-data() -> ()  [unwired: 7 out]
        n714 = xnode "Read/Write Control"("FPGA VI Reference In"=w1035, "Cont. Scan"="Continuous AOD Scanning") -> ("error out"=w1037:errorcluster)  [unwired: 1 in, 1 out]
      }
      event "Index": Value Change {
        n715 = event-data() -> ()  [unwired: 7 out]
        n716 = call "Create new save file.vi"("Insert"="", "Ext"=".dat" ("string"), "Index In"="Index") -> ("Path Out"=→"Save file name":path, "Index Out"=w1038:dbl)
        "Save index" <- w1038
        n717 = local write "Index"(w1038) -> ()
      }
      event "AO1", "AO2": Value Change {
        w1052 = 10.0 ("y")
        w1051 = 32767.0 ("y")
        n718 = event-data() -> ()  [unwired: 7 out]
        n719 = local read "AO2"() -> (w1050:dbl)
        n720 = local read "AO1"() -> (w1047:dbl)
        n721 = Multiply(x=w1047, y=w1051) -> (x*y=w1046:dbl)
        n722 = Multiply(x=w1050, y=w1051) -> (x*y=w1049:dbl)
        n723 = Divide(x=w1046, y=w1052) -> (x/y=w1045:dbl)
        n724 = Divide(x=w1049, y=w1052) -> (x/y=w1048:dbl)
        n725 = To Word Integer(number=w1045) -> (16bit integer=w1053:i16)
        n726 = To Word Integer(number=w1048) -> (16bit integer=w1054:i16)
        n727 = xnode "Read/Write Control"("FPGA VI Reference In"=w1043, "AO1"=w1053, "AO2"=w1054) -> ("error out"=w1044:errorcluster)  [unwired: 1 in, 1 out]
      }
      event "Inject Pump 1": Value Change {
        n728 = event-data() -> ()  [unwired: 7 out]
        n729 = local read "Use Harvard pumps\nfor beads (else Chemyx)"() -> (w1056:bool)
        n730 = case shown="True" w1056 {
          tunnel: "Inject Pump 1" -> [w1060 w1098]
          tunnel: w1055 -> [_ w1099]
          frame False {
            n731 = local read "Pump write delay (ms)"() -> (w1059:dbl)
            n732 = local read "Chemyx Syringe Pump Serial Port"() -> (w1058:refnum<visa-resource-name>)
            n733 = case shown="True" w1060 {
              tunnel: w1059 -> [w1066 w1080]
              tunnel: w1058 -> [w1063 w1079]
              frame False {
                n734 = flat-sequence {
                  tunnel: w1063 -> [w1067]
                  tunnel: [w1067] -> w1064
                  tunnel: w1066 -> [_]
                  tunnel: [w1070] -> w1065
                  tunnel: w1064 -> [w1070]
                  tunnel: w1065 -> [w1071]
                  tunnel: [w1071] -> w1061
                  tunnel: [w1073] -> w1062
                  tunnel: w1061 -> [w1073]
                  tunnel: w1062 -> [w1075]
                  frame #0 {
                    n735 = call "Write to pump.vi"("string"="enter pump1", "VISA resource name"=w1067) -> ()  [unwired: 1 out]
                  }
                  frame #1 {
                    n736 = Wait (ms)(milliseconds to wait="Pump pause delay (ms)") -> ()  [unwired: 1 out]
                  }
                  frame #2 {
                    n737 = call "Write to pump.vi"("string"="stop", "VISA resource name"=w1071) -> ()  [unwired: 1 out]
                  }
                  frame #3 {
                    n738 = Wait (ms)(milliseconds to wait=u32 500) -> ()  [unwired: 1 out]
                  }
                  frame #4 {
                    n739 = call "Write to pump.vi"("string"="stop", "VISA resource name"=w1075) -> ()  [unwired: 1 out]
                  }
                }
              }
              frame True {
                n740 = flat-sequence {
                  tunnel: w1079 -> [w1089]
                  tunnel: w1080 -> [w1084]
                  tunnel: w1080 -> [w1091]
                  tunnel: w1079 -> [w1092]
                  tunnel: [w1092] -> w1077
                  tunnel: [w1094] -> w1078
                  tunnel: w1077 -> [w1094]
                  tunnel: w1078 -> [w1096]
                  frame #0 {
                    n741 = local read "All Pump Parameters"() -> (w1083:T5)
                    n742 = Unbundle By Name(w1083) -> ("Pump 1"=w1090:T30)
                    n743 = call "Set pump parameters.vi"("Pump write delay (ms)"=w1084, "Volume (uL)"="Ch 1 Inject Volume (uL)", "Rate (uL/h)"="Ch 1 Inject Rate (ul/h)", "Units"=4.0, "Pump #"=1.0, "Pump Parameters In"=w1090, "VISA resource name"=w1089) -> ("Pump Parameters Out"=w1082:T30)  [unwired: 3 in]
                    n744 = Bundle By Name(cluster=w1083, "Pump 1"=w1082) -> (w1081:T5)
                    n745 = local write "All Pump Parameters"(w1081) -> ()
                  }
                  frame #1 {
                    n746 = Wait (ms)(milliseconds to wait=w1091) -> ()  [unwired: 1 out]
                  }
                  frame #2 {
                    n747 = call "Write to pump.vi"("string"="start", "VISA resource name"=w1092) -> ()  [unwired: 1 out]
                  }
                  frame #3 {
                    n748 = Wait (ms)(milliseconds to wait=u32 500) -> ()  [unwired: 1 out]
                  }
                  frame #4 {
                    n749 = call "Write to pump.vi"("string"="start", "VISA resource name"=w1096) -> ()  [unwired: 1 out]
                  }
                }
              }
            }
          }
          frame True {
            n750 = case shown="False" w1098 {
              tunnel: w1099 -> [w1100 w1110]
              frame False {
                n751 = flat-sequence {
                  tunnel: w1100 -> [w1102]
                  frame #0 {
                    n752 = local write "Flushing P1"(FALSE ("Flushing P1")) -> ()
                    n753 = Concatenate Strings("stop" ("string"), "\r") -> (w1104:string)
                    n754 = VISA Write(VISA resource name=w1102, write buffer=w1104) -> ()  [unwired: 1 in, 3 out]
                  }
                  frame #1 {
                    n755 = property on="Clear Volume P1" class="Bool (strict)"("Val(Sgnl)"=TRUE ("Value (Signaling)")) -> ()  [unwired: 2 in, 2 out]
                  }
                }
              }
              frame True {
                n756 = local read "Normal Flow Rate (ul/h) P1"() -> (w1108:dbl)
                n757 = Number To Decimal String(number=w1108) -> (decimal integer string=w1114:string)  [unwired: 1 in]
                n758 = Concatenate Strings("irate  " ("string"), w1114, " u/h" ("string"), "\r") -> (w1112:string)
                n759 = VISA Write(VISA resource name=w1110, write buffer=w1112) -> (VISA resource name out=w1109:refnum<visa-resource-name>)  [unwired: 1 in, 2 out]
                n760 = Concatenate Strings("irun" ("string"), "\r") -> (w1116:string)
                n761 = VISA Write(VISA resource name=w1109, write buffer=w1116) -> ()  [unwired: 1 in, 3 out]
              }
            }
          }
        }
      }
      event "Inject Pump 3": Value Change {
        n762 = event-data() -> ()  [unwired: 7 out]
        n763 = local read "Use Harvard pumps\nfor beads (else Chemyx)"() -> (w1119:bool)
        n764 = case shown="True" w1119 {
          tunnel: "Inject Pump 3" -> [w1123 w1162]
          tunnel: w1118 -> [_ w1161]
          frame False {
            n765 = local read "Pump write delay (ms)"() -> (w1122:dbl)
            n766 = case shown="True" w1123 {
              tunnel: w1122 -> [w1129 w1143]
              tunnel: "Chemyx Syringe Pump Serial Port" -> [w1126 w1142]
              frame False {
                n767 = flat-sequence {
                  tunnel: w1126 -> [w1130]
                  tunnel: [w1130] -> w1127
                  tunnel: w1129 -> [_]
                  tunnel: [w1133] -> w1128
                  tunnel: w1127 -> [w1133]
                  tunnel: w1128 -> [w1134]
                  tunnel: [w1134] -> w1124
                  tunnel: [w1136] -> w1125
                  tunnel: w1124 -> [w1136]
                  tunnel: w1125 -> [w1138]
                  frame #0 {
                    n768 = call "Write to pump.vi"("string"="enter pump3", "VISA resource name"=w1130) -> ()  [unwired: 1 out]
                  }
                  frame #1 {
                    n769 = local read "Pump pause delay (ms)"() -> (w1132:u32)
                    n770 = Wait (ms)(milliseconds to wait=w1132) -> ()  [unwired: 1 out]
                  }
                  frame #2 {
                    n771 = call "Write to pump.vi"("string"="stop", "VISA resource name"=w1134) -> ()  [unwired: 1 out]
                  }
                  frame #3 {
                    n772 = Wait (ms)(milliseconds to wait=u32 0) -> ()  [unwired: 1 out]
                  }
                  frame #4 {
                    n773 = call "Write to pump.vi"("string"="stop", "VISA resource name"=w1138) -> ()  [unwired: 1 out]
                  }
                }
              }
              frame True {
                n774 = flat-sequence {
                  tunnel: w1142 -> [w1152]
                  tunnel: w1143 -> [w1147]
                  tunnel: w1143 -> [w1154]
                  tunnel: w1142 -> [w1155]
                  tunnel: [w1155] -> w1141
                  tunnel: [w1158] -> w1140
                  tunnel: w1141 -> [w1158]
                  tunnel: w1140 -> [w1159]
                  frame #0 {
                    n775 = local read "All Pump Parameters"() -> (w1146:T5)
                    n776 = Unbundle By Name(w1146) -> ("Pump 3"=w1153:T30)
                    n777 = call "Set pump parameters.vi"("Pump write delay (ms)"=w1147, "Volume (uL)"="Ch 3 Inject Volume (uL)", "Rate (uL/h)"="Ch 3 Inject Rate (ul/h)", "Units"=4.0, "Pump #"=3.0, "Pump Parameters In"=w1153, "VISA resource name"=w1152) -> ("Pump Parameters Out"=w1145:T30)  [unwired: 3 in]
                    n778 = Bundle By Name(cluster=w1146, "Pump 3"=w1145) -> (w1144:T5)
                    n779 = local write "All Pump Parameters"(w1144) -> ()
                  }
                  frame #1 {
                    n780 = Wait (ms)(milliseconds to wait=w1154) -> ()  [unwired: 1 out]
                  }
                  frame #2 {
                    n781 = call "Write to pump.vi"("string"="start", "VISA resource name"=w1155) -> ()  [unwired: 1 out]
                  }
                  frame #3 {
                    n782 = Wait (ms)(milliseconds to wait=u32 500) -> ()  [unwired: 1 out]
                  }
                  frame #4 {
                    n783 = call "Write to pump.vi"("string"="start", "VISA resource name"=w1159) -> ()  [unwired: 1 out]
                  }
                }
              }
            }
          }
          frame True {
            n784 = case shown="False" w1162 {
              tunnel: w1161 -> [w1163 w1170]
              frame False {
                n785 = flat-sequence {
                  tunnel: w1163 -> [w1165]
                  frame #0 {
                    n786 = local write "Flushing P3"(FALSE ("Flushing P3")) -> ()
                    n787 = Concatenate Strings("stop" ("string"), "\r") -> (w1167:string)
                    n788 = VISA Write(VISA resource name=w1165, write buffer=w1167) -> ()  [unwired: 1 in, 3 out]
                  }
                  frame #1 {
                    n789 = property on="Clear Volume P3" class="Bool (strict)"("Val(Sgnl)"=TRUE ("Value (Signaling)")) -> ()  [unwired: 2 in, 2 out]
                  }
                }
              }
              frame True {
                n790 = local read "Normal Flow Rate (ul/h) P3"() -> (w1171:dbl)
                n791 = Number To Decimal String(number=w1171) -> (decimal integer string=w1177:string)  [unwired: 1 in]
                n792 = Concatenate Strings("irate  " ("string"), w1177, " u/h" ("string"), "\r") -> (w1175:string)
                n793 = VISA Write(VISA resource name=w1170, write buffer=w1175) -> (VISA resource name out=w1173:refnum<visa-resource-name>)  [unwired: 1 in, 2 out]
                n794 = Concatenate Strings("irun" ("string"), "\r") -> (w1179:string)
                n795 = VISA Write(VISA resource name=w1173, write buffer=w1179) -> ()  [unwired: 1 in, 3 out]
              }
            }
          }
        }
      }
      event "Inject Pump 2": Value Change {
        n796 = event-data() -> ()  [unwired: 7 out]
        n797 = local read "Pump write delay (ms)"() -> (w1183:dbl)
        n798 = flat-sequence {
          tunnel: w1181 -> [w1196]
          tunnel: w1183 -> [w1192]
          tunnel: "Inject Pump 2" -> [_]
          tunnel: w1183 -> [w1198]
          tunnel: w1181 -> [w1199]
          frame #0 {
            n799 = local read "All Pump Parameters"() -> (w1191:T5)
            n800 = Multiply(x=60.0, y="Flush Center Ch Rate (ul/m)") -> (x*y=w1188:dbl)
            n801 = Unbundle By Name(w1191) -> ("Pump 2"=w1197:T30)
            n802 = call "Set pump parameters.vi"("Pump write delay (ms)"=w1192, "Volume (uL)"="Flush Center Ch Volume (uL)", "Rate (uL/h)"=w1188, "Units"=3.0, "Pump #"=2.0, "Pump Parameters In"=w1197, "VISA resource name"=w1196) -> ("Pump Parameters Out"=w1190:T30)  [unwired: 3 in]
            n803 = Bundle By Name(cluster=w1191, "Pump 2"=w1190) -> (w1189:T5)
            n804 = local write "All Pump Parameters"(w1189) -> ()
            n805 = Add(x="Flush Center Ch Volume (uL)", y="Total Volume\nFlushed (uL)") -> (x+y=w1185:dbl)
            n806 = local write "Total Volume\nFlushed (uL)"(w1185) -> ()
          }
          frame #1 {
            n807 = Wait (ms)(milliseconds to wait=w1198) -> ()  [unwired: 1 out]
          }
          frame #2 {
            n808 = call "Write to pump.vi"("string"="start", "VISA resource name"=w1199) -> ()  [unwired: 1 out]
          }
        }
        n809 = local read "Chemyx Syringe Pump Serial Port"() -> (w1181:refnum<visa-resource-name>)
      }
      event "Sample Channel\nFlow": Value Change {
        n810 = event-data() -> ()  [unwired: 7 out]
        n811 = Select(t="irun" ("string"), s="Sample Channel\nFlow", f="stop" ("string")) -> (s? t:f=w1203:string)
        n812 = Concatenate Strings(w1203, "\r") -> (w1206:string)
        n813 = VISA Write(VISA resource name=w1201, write buffer=w1206) -> ()  [unwired: 1 in, 3 out]
      }
      event "Start Flow": Value Change {
        n814 = event-data() -> ()  [unwired: 7 out]
        n815 = local write "Sample Channel\nFlow"(TRUE ("Sample Channel\nFlow")) -> ()
        n816 = local write "Start Flow"(FALSE ("Start Flow")) -> ()
        n817 = Concatenate Strings("irun" ("string"), "\r") -> (w1212:string)
        n818 = VISA Write(VISA resource name=w1208, write buffer=w1212) -> ()  [unwired: 1 in, 3 out]
      }
      event "Stop Flow": Value Change {
        w1214 = FALSE ("Stop Flow")
        n819 = event-data() -> ()  [unwired: 7 out]
        n820 = local write "Stop Flow"(w1214) -> ()
        n821 = local write "Sample Channel\nFlow"(w1214) -> ()
        n822 = Concatenate Strings("stop" ("string"), "\r") -> (w1217:string)
        n823 = VISA Write(VISA resource name=w1215, write buffer=w1217) -> ()  [unwired: 1 in, 3 out]
      }
      event "Flow rate (uL/h)": Value Change {
        n824 = event-data() -> ()  [unwired: 7 out]
        n825 = Number To Decimal String(number="Flow rate (uL/h)") -> (decimal integer string=w1224:string)  [unwired: 1 in]
        n826 = Concatenate Strings("irate  " ("string"), w1224, " u/h" ("string"), "\r") -> (w1223:string)
        n827 = VISA Write(VISA resource name=w1220, write buffer=w1223) -> ()  [unwired: 1 in, 3 out]
      }
      event "Flush Sample": Value Change {
        n828 = event-data() -> ()  [unwired: 7 out]
        n829 = flat-sequence {
          tunnel: w1229 -> [w1257]
          tunnel: [w1237] -> w1228
          tunnel: [w1231] -> w1226
          tunnel: w1228 -> [w1261]
          tunnel: [w1261] -> w1227
          tunnel: w1226 -> [w1260]
          tunnel: w1227 -> [w1266]
          frame #0 {
            # "set paramaters (rate, volume) for flush, clear volume"
            n830 = Number To Decimal String(number="Flush rate (uL/m)") -> (decimal integer string=w1253:string)  [unwired: 1 in]
            n831 = Concatenate Strings("irate  " ("string"), w1253, " u/m" ("string"), "\r") -> (w1255:string)
            n832 = VISA Write(VISA resource name=w1257, write buffer=w1255) -> (VISA resource name out=w1251:refnum<visa-resource-name>)  [unwired: 1 in, 2 out]
            n833 = Reciprocal(x="Flush rate (uL/m)") -> (1/x=w1234:dbl)
            n834 = Number To Decimal String(number="Volume (uL)") -> (decimal integer string=w1242:string)  [unwired: 1 in]
            n835 = Multiply(x="Volume (uL)", y=w1234) -> (x*y=w1233:dbl)
            n836 = Concatenate Strings("tvolume  " ("string"), w1242, " u" ("string"), "\r") -> (w1240:string)
            n837 = Multiply(x=w1233, y=60000.0) -> (x*y=w1231:dbl)
            n838 = VISA Write(VISA resource name=w1251, write buffer=w1240) -> (VISA resource name out=w1239:refnum<visa-resource-name>)  [unwired: 1 in, 2 out]
            n839 = Concatenate Strings("cvolume" ("string"), "\r") -> (w1238:string)
            n840 = VISA Write(VISA resource name=w1239, write buffer=w1238) -> (VISA resource name out=w1249:refnum<visa-resource-name>)  [unwired: 1 in, 2 out]
            n841 = Concatenate Strings("irun" ("string"), "\r") -> (w1247:string)
            n842 = VISA Write(VISA resource name=w1249, write buffer=w1247) -> (VISA resource name out=w1237:refnum<visa-resource-name>)  [unwired: 1 in, 2 out]
          }
          frame #1 {
            # "Have to wait until\nflow is done to reset\nrate"
            n843 = Add(x=w1260, y=100.0) -> (x+y=w1259:dbl)
            n844 = Wait (ms)(milliseconds to wait=w1259) -> ()  [unwired: 1 out]
          }
          frame #2 {
            # "reset flow rate to usual flow rate"
            n845 = local read "Flow rate (uL/h)"() -> (w1272:dbl)
            n846 = Number To Decimal String(number=w1272) -> (decimal integer string=w1270:string)  [unwired: 1 in]
            n847 = Concatenate Strings("irate  " ("string"), w1270, " u/h" ("string"), "\r") -> (w1268:string)
            n848 = VISA Write(VISA resource name=w1266, write buffer=w1268) -> (VISA resource name out=w1262:refnum<visa-resource-name>)  [unwired: 1 in, 2 out]
            n849 = Concatenate Strings("cvolume" ("string"), "\r") -> (w1263:string)
            n850 = VISA Write(VISA resource name=w1262, write buffer=w1263) -> ()  [unwired: 1 in, 3 out]
          }
        }
      }
      event "Flush Pump 3": Value Change {
        n851 = event-data() -> ()  [unwired: 7 out]
        n852 = flat-sequence {
          tunnel: w1273 -> [w1276]
          frame #0 {
            # "set paramaters (rate, volume) for flush, clear volume"
            n853 = Number To Decimal String(number="Flush rate (uL/m) P3") -> (decimal integer string=w1298:string)  [unwired: 1 in]
            n854 = local write "Inject Pump 3"(TRUE ("Inject Pump 3")) -> ()
            n855 = Concatenate Strings("irate  " ("string"), w1298, " u/m" ("string"), "\r") -> (w1300:string)
            n856 = VISA Write(VISA resource name=w1276, write buffer=w1300) -> (VISA resource name out=w1296:refnum<visa-resource-name>)  [unwired: 1 in, 2 out]
            n857 = Reciprocal(x="Flush rate (uL/m) P3") -> (1/x=w1280:dbl)
            n858 = Number To Decimal String(number="Volume (uL) P3") -> (decimal integer string=w1287:string)  [unwired: 1 in]